vi "UHR-Fleezers Control (host) - 12.8.vi"() -> ()   [LabVIEW 2012] (continued)
          tunnel: [w4443 w4464] -> w4429
          tunnel: [w4442 w4463] -> w4428
          tunnel: w4427 -> [w4443 w4469]
          tunnel: w4426 -> [w4442 w4472]
          tunnel: w4423 -> [_ _]
          frame False {
            w4444 = TRUE ("AI to FIFO")
            n2524 = xnode "Read/Write Control"("FPGA VI Reference In"=w4448, "error in"=w4447, "AI to FIFO"=w4444, "APD to FIFO"=w4444, "Start scan (MCL)"=w4444) -> ("FPGA VI Reference Out"=w4446:T20, "error out"=w4445:errorcluster)
          }
          frame True {
            w4476 = TRUE ("AI to FIFO")
            n2525 = local read "Scan steps (MCL)"() -> (w4455:u64)
            n2526 = local read "Scan lines (y)"() -> (w4451:u64)
            n2527 = local read "Fast Scan Dir"() -> (w4462:bool)
            n2528 = local read "Actual MCL Inc (V)"() -> (w4452:dbl)
            n2529 = Decrement(x=w4451) -> (x-1=w4450:u64)
            n2530 = Decrement(x=w4455) -> (x-1=w4454:u64)
            n2531 = Multiply(x=w4452, y=w4450) -> (x*y=w4449:dbl)
            n2532 = Divide(x=w4449, y=2.0) -> (x/y=w4459:dbl)
            n2533 = Multiply(x=w4452, y=w4454) -> (x*y=w4453:dbl)
            n2534 = Divide(x=w4453, y=2.0) -> (x/y=w4458:dbl)
            n2535 = Select(t=w4458, s=w4462, f=w4459) -> (s? t:f=w4457:dbl)
            n2536 = Select(t=w4459, s=w4462, f=w4458) -> (s? t:f=w4461:dbl)
            n2537 = Subtract(x=w4469, y=w4461) -> (x-y=w4460:dbl)
            n2538 = Subtract(x=w4472, y=w4457) -> (x-y=w4456:dbl)
            n2539 = local read "2D or 1D Scan"() -> (w4474:bool)
            n2540 = Not(x=w4462) -> (.not. x?=w4468:bool)
            n2541 = Not(x=w4474) -> (.not. x?=w4470:bool)
            n2542 = And(x=w4462, y=w4470) -> (x .and. y?=w4471:bool)
            n2543 = And(x=w4470, y=w4468) -> (x .and. y?=w4473:bool)
            n2544 = Select(t=w4472, s=w4473, f=w4456) -> (s? t:f=w4463:dbl)
            n2545 = Select(t=w4469, s=w4471, f=w4460) -> (s? t:f=w4464:dbl)
            n2546 = call "Volt to I16.vi"("Voltage In"=w4464) -> ("I16 Voltage Out"=w4467:i16)
            n2547 = call "Volt to I16.vi"("Voltage In"=w4463) -> ("I16 Voltage Out"=w4466:i16)
            n2548 = xnode "Read/Write Control"("FPGA VI Reference In"=w4480, "error in"=w4479, "AI to FIFO"=w4476, "APD to FIFO"=w4476, "Start scan (MCL)"=w4476, "AO1"=w4467, "AO2"=w4466) -> ("FPGA VI Reference Out"=w4478:T20, "error out"=w4477:errorcluster)
          }
        }
        "Initial Y" <- w4429
        "Initial X" <- w4428
        n2549 = local write "Tab Control 6"(T3."Imaging" ("Tab Control 6")) -> ()
        "wait to reset values" <- w4430
      }
    }
    n2550 = local read "APD Elements/DMA read"() -> (w3570:u32)
    n2551 = local read "Trap AI Elements/DMA read"() -> (w3785:u32)
    n2552 = xnode "Get APD Data"("FPGA VI Reference In"=w3726, "error in"=w3725, "Number of Elements"=w3570, "Timeout (ms)"=-1) -> ("Data"=w3756:u32[], "Elements Remaining"=→"APD FIFO Elements Remaining":u32)  [unwired: 2 out]
    n2553 = local read "Trap Pos Elements/DMA read"() -> (w3722:u32)
    n2554 = xnode "Invoke Method"("FPGA VI Reference In"=w3726, "error in"=w3725, "Number of Elements"=w3722, "Timeout (ms)"=-1) -> ("Data"=w3686:u16[], "Elements Remaining"=→"Trap Pos FIFO El Remaining":u32)  [unwired: 2 out]
    n2555 = xnode "Get Trap Data"("FPGA VI Reference In"=w3726, "error in"=w3725, "Number of Elements"=w3785, "Timeout (ms)"=-1 ("Timeout")) -> ("FPGA VI Reference Out"=w3621:T20, "error out"=w3620:errorcluster, "Data"=w3687:i16[], "Elements Remaining"=w3903:u32)
    "FIFO El. Rem." <- w3903
    n2556 = local read "DMA Update Period (s)"() -> (w3786:dbl)
    n2557 = local read "Trap AI FIFO Depth"() -> (w3905:u32)
    n2558 = local read "Number of APDs"() -> (w3589:u8)
    n2559 = Decimate 1D Array(w3686) -> (w3683:u16[], w3685:u16[], w3684:u16[])
    n2560 = feedback #6(0.0) -> (w3715:dbl)
    n2561 = Add(x=w3786, y=w3715) -> (x+y=w3879:dbl)
    n2562 = feedback-in #6(w3879) -> ()
    n2563 = To Time Stamp(1:w3715) -> (0:w3714:timestamp)
    n2564 = Subtract(x=w3905, y=w3785) -> (x-y=w3904:u32)
    n2565 = To Unsigned Long Integer(number=w3683) -> (unsigned 32bit integer=w3682:u32[])
    n2566 = Join Numbers(hi=w3685, lo=w3684) -> ((hi.lo)=w3681:u32[])
    n2567 = Divide(x=w3903, y=w3904) -> (x/y=w3902:dbl)
    "Buffer Status" <- w3902
    n2568 = case "Deinterlace APD signals" shown="3, Default" w3589 {
      tunnel: [w3929 w3935] -> w3569
      tunnel: w3756 -> [w3930 w3934]
      tunnel: [w3928 w3933] -> w3568
      tunnel: [w3927 w3931] -> w3557
      frame 3, Default {
        n2569 = Decimate 1D Array "APD signals"(w3930) -> (w3929:u32[], w3928:u32[], w3927:u32[])
      }
      frame 2 {
        n2570 = Decimate 1D Array "APD signals"(w3934) -> (w3935:u32[], w3933:u32[])
        n2571 = Multiply(x=w3933, y=u32 0) -> (x*y=w3931:u32[])
      }
    }
    n2572 = Join Numbers(hi=w3682, lo=w3681) -> ((hi.lo)=w3675:u64[])
    n2573 = call "IR AOM word to freq - vec.vi"("Frequency Word In (double vec)"=w3675) -> ("Frequency Out"=w3721:dbl[])
    n2574 = Equal?(x=w3902, y=1.0) -> (x = y?=w3900:bool)
    n2575 = case "Alert buffer overflow" shown="True" w3900 {
      frame False {
      }
      frame True {
        n2576 = call <vilib>:"Beep.vi"() -> ()  [unwired: 3 in, 9 out]
        "Overflow (data lost)" <- TRUE ("Overflow (data lost)")
      }
    }
    n2577 = Decimate 1D Array(w3721) -> (w3720:dbl[], w3719:dbl[])
    n2578 = Build Array(w3720, w3719) -> (w3718:dbl[][])
    n2579 = Bundle(w3569, w3568, w3557) -> (w3573:cluster{u32[], u32[], u32[]})  [unwired: 1 in]
    n2580 = Build Array(w3569, w3568, w3557) -> (w3840:u32[][])
    n2581 = for {
      tunnel: w3569 -> [w3925] mode=indexing
      n2582 = call "Smart Buffer (DBL) 1.vi"("new element [write]"=w3925, "mode"=T21."write") -> ()  [unwired: 4 in, 6 out]
    }
    n2583 = local read "APD Integration Time (s)"() -> (w3584:dbl)
    n2584 = To Double Precision Float(number=w3840) -> (double precision float=w3841:dbl[][])
    n2585 = feedback #7 "APD3"(w3557) -> (w3558:u32[])
    n2586 = feedback #8 "APD2"(w3568) -> (w3744:u32[])
    n2587 = feedback #9 "APD1"(w3569) -> (w3839:u32[])
    n2588 = Build Array (concatenate)(w3744, w3568) -> (w3743:u32[])
    n2589 = Build Array (concatenate)(w3558, w3557) -> (w3556:u32[])
    n2590 = Build Array (concatenate)(w3839, w3569) -> (w3836:u32[])
    n2591 = for {
      tunnel: w3568 -> [w3924] mode=indexing
      n2592 = call "Smart Buffer (DBL) 2.vi"("new element [write]"=w3924, "mode"=T21."write") -> ()  [unwired: 4 in, 6 out]
    }
    n2593 = Array Size(array=w3836) -> (size(s)=w3833:i32)
    n2594 = Array Size(array=w3569) -> (size(s)=w3835:i32)
    n2595 = Multiply(x=w3835, y="APD Ave N") -> (x*y=w3834:dbl)
    n2596 = Greater?(x=w3833, y=w3834) -> (0:w3837:bool)
    n2597 = Bundle("APD 1", "APD 2", "APD 3") -> (w3873:cluster{string, string, string})  [unwired: 1 out]
    n2598 = local read "Trap Sets"() -> (w3784:u32)
    n2599 = case shown="True" w3837 {
      tunnel: w3836 -> [w4236 w4245]
      tunnel: [w4236 w4243] -> w3791
      tunnel: w3834 -> [_ w4238]
      tunnel: w3833 -> [_ w4244]
      tunnel: w3743 -> [w4235 w4242]
      tunnel: [w4235 w4241] -> w3741
      tunnel: w3556 -> [w4234 w4240]
      tunnel: [w4234 w4237] -> w3585
      frame False {
      }
      frame True {
        n2600 = Subtract(x=w4244, y=w4238) -> (x-y=w4239:dbl)
        n2601 = Array Subset "APD3"(array=w4240, index=w4239, length=w4238) -> (w4237:u32[])
        n2602 = Array Subset "APD2"(array=w4242, index=w4239, length=w4238) -> (w4241:u32[])
        n2603 = Array Subset "APD1"(array=w4245, index=w4239, length=w4238) -> (w4243:u32[])
      }
    }
    n2604 = feedback-in #7(w3585) -> ()
    n2605 = feedback-in #8(w3741) -> ()
    n2606 = feedback-in #9(w3791) -> ()
    n2607 = Cluster To Array(cluster=w3873) -> (array=w3870:string[])
    n2608 = for "APD" {
      tunnel: w3841 -> [w4492] mode=indexing
      tunnel: w3584 -> [w4499]
      tunnel: [w4495] -> w3745 mode=indexing
      tunnel: "APD Disp. Scale" -> [w4496]
      tunnel: w3870 -> [w4494] mode=indexing
      tunnel: "APD Disp. Downsample" -> [w4490]
      tunnel: [w4493] -> w3869
      workers-P: _ -> [_]
      tunnel: w3714 -> [w4489]
      n2609 = call "integrate 1D array interval - double.vi"("Ave N"=w4490, "Array In"=w4492) -> ("Array Out"=w4491:dbl[])  [unwired: 1 out]
      n2610 = Multiply(x=w4499, y=w4490) -> (x*y=w4493:dbl)
      n2611 = Divide(x=w4491, y=w4496) -> (x/y=w4497:dbl[])
      n2612 = Bundle By Name("t0"=w4489, "Y"=w4497, "dt"=w4493) -> (w4498:waveform(dbl))  [unwired: 1 out]
      n2613 = Set Waveform Attribute(5:w4494, 6:"NI_ChannelName" ("name"), 7:w4498) -> (3:w4495:waveform(dbl))  [unwired: 1 in, 2 out]
    }
    "APD Display Period (s)" <- w3869
    n2614 = Reciprocal(x=w3869) -> (1/x=→"APD Display Freq. (Hz)":dbl)
    n2615 = case "Deinterlace trap data, average down PSD" shown="2" w3784 {
      tunnel: w3687 -> [w4517 w4582]
      tunnel: [w4514 w4579] -> w3777
      tunnel: [w4517 w4581] -> w3678
      tunnel: "Detector Type" -> [w4516 w4577]
      tunnel: [w4515 w4580] -> w3776
      tunnel: [w4513 w4578] -> w3877
      frame 1, Default {
        n2616 = Divide(x=w4517, y=3276.7) -> (x/y=w4518:dbl[])
        n2617 = Decimate 1D Array(w4518) -> (w4527:dbl[], w4526:dbl[], w4525:dbl[], w4524:dbl[], w4523:dbl[], w4522:dbl[], w4521:dbl[], w4520:dbl[])
        n2618 = case shown="\"IR-QPD + PSD + FB-QPD position\"" w4516 {
          tunnel: w4527 -> [w4551 w4576]
          tunnel: w4526 -> [w4550 w4575]
          tunnel: w4525 -> [w4535 w4553]
          tunnel: w4524 -> [w4536 w4563]
          tunnel: w4523 -> [w4549 w4574]
          tunnel: w4522 -> [w4548 w4573]
          tunnel: w4521 -> [w4532 w4554]
          tunnel: w4520 -> [w4531 w4552]
          tunnel: [w4530 w4560] -> w4515
          tunnel: [w4529 w4559] -> w4514
          tunnel: [w4528 w4558] -> w4513
          frame "IR-QPD + PSD + FB-QPD", Default {
            w4528 = 0  # Channel pattern
            n2619 = Divide(x=w4551, y=w4536) -> (x/y=w4538:dbl[])
            n2620 = Divide(x=w4550, y=w4536) -> (x/y=w4537:dbl[])
            n2621 = Divide(x=w4549, y=w4532) -> (x/y=w4534:dbl[])
            n2622 = Divide(x=w4548, y=w4531) -> (x/y=w4533:dbl[])
            n2623 = Build Array(w4538, w4537, w4536, w4535, w4534, w4533, w4532, w4531) -> (w4529:dbl[][])
            n2624 = Bundle("T1 Y", "T1 X", "T1 Sum", "FB Sum", "PSD Y", "PSD X", "PSD Y Sum", "PSD X Sum") -> (w4547:T44)  [unwired: 1 out]
            n2625 = Cluster To Array(cluster=w4547) -> (array=w4530:string[])
          }
          frame "IR-QPD + PSD + FB-QPD position" {
            w4558 = 3  # Channel pattern
            n2626 = Negate(x=w4554) -> (-x=w4555:dbl[])
            n2627 = Divide(x=w4576, y=w4563) -> (x/y=w4565:dbl[])
            n2628 = Divide(x=w4575, y=w4563) -> (x/y=w4564:dbl[])
            n2629 = Divide(x=w4574, y=w4554) -> (x/y=w4562:dbl[])
            n2630 = Divide(x=w4573, y=w4555) -> (x/y=w4561:dbl[])
            n2631 = Build Array(w4565, w4564, w4563, w4552, w4553, w4562, w4561, w4554) -> (w4559:dbl[][])
            n2632 = Bundle("T1 Y", "T1 X", "T1 Sum", "FB X", "FB Sum", "PSD Y", "PSD X", "PSD Y Sum") -> (w4572:T44)  [unwired: 1 out]
            n2633 = Cluster To Array(cluster=w4572) -> (array=w4560:string[])
          }
        }
      }
      frame 2 {
        n2634 = case shown="\"IR-QPD + PSD + FB-QPD X position\", Default" w4577 {
          tunnel: w4582 -> [w4644 w4716 w4787]
          tunnel: [w4583 w4707 w4718] -> w4581
          tunnel: [w4610 w4698 w4765] -> w4580
          tunnel: [w4609 w4661 w4732] -> w4579
          tunnel: [w4603 w4696 w4763] -> w4578
          frame "IR-QPD + PSD + FB-QPD" {
            w4603 = 1  # Channel pattern
            # "time average x2 the 4th signal and the 4 psd signals (detection laser)"
            # "deinterlace 3 signals from qpd"
            n2635 = Decimate 1D Array(w4644) -> (w4643:i16[], w4642:i16[], w4608:i16[], w4641:i16[], w4631:i16[], w4629:i16[], w4628:i16[], w4626:i16[])
            n2636 = Decimate 1D Array(w4608) -> (w4607:i16[], w4606:i16[])
            n2637 = Decimate 1D Array(w4643) -> (w4640:i16[], w4612:i16[])
            n2638 = Decimate 1D Array(w4642) -> (w4639:i16[], w4637:i16[])
            n2639 = Decimate 1D Array(w4641) -> (w4638:i16[], w4636:i16[])
            n2640 = call "downsample 1D array - double.vi"("Ave N"=2.0, "Array In"=w4631) -> ("Array Out"=w4630:dbl[])  [unwired: 1 out]
            n2641 = call "downsample 1D array - double.vi"("Ave N"=2.0, "Array In"=w4629) -> ("Array Out"=w4611:dbl[])  [unwired: 1 out]
            n2642 = call "downsample 1D array - double.vi"("Ave N"=2.0, "Array In"=w4628) -> ("Array Out"=w4627:dbl[])  [unwired: 1 out]
            n2643 = call "downsample 1D array - double.vi"("Ave N"=2.0, "Array In"=w4626) -> ("Array Out"=w4625:dbl[])  [unwired: 1 out]
            n2644 = Interleave 1D Arrays(w4640, w4639, w4638, w4612, w4637, w4636, w4607, w4606, w4630, w4611, w4627, w4625) -> (w4624:dbl[])
            n2645 = Divide(x=w4624, y=3276.7) -> (x/y=w4623:dbl[])
            n2646 = Decimate 1D Array(w4623) -> (w4622:dbl[], w4621:dbl[], w4620:dbl[], w4619:dbl[], w4618:dbl[], w4617:dbl[], w4605:dbl[], w4604:dbl[], w4616:dbl[], w4615:dbl[], w4614:dbl[], w4613:dbl[])
            n2647 = Divide(x=w4622, y=w4620) -> (x/y=w4590:dbl[])
            n2648 = Divide(x=w4621, y=w4620) -> (x/y=w4589:dbl[])
            n2649 = Divide(x=w4619, y=w4617) -> (x/y=w4588:dbl[])
            n2650 = Divide(x=w4618, y=w4617) -> (x/y=w4587:dbl[])
            n2651 = Divide(x=w4616, y=w4614) -> (x/y=w4586:dbl[])
            n2652 = Divide(x=w4615, y=w4613) -> (x/y=w4585:dbl[])
            n2653 = Build Array(w4590, w4589, w4620, w4588, w4587, w4617, w4605, w4604, w4586, w4585, w4614, w4613) -> (w4609:dbl[][])
            n2654 = Bundle("T1 Y", "T1 X", "T1 Sum", "T2 Y", "T2 X", "T2 Sum", "T1 FB Sum", "T2 FB Sum", "PSD Y", "PSD X", "PSD Y Sum", "PSD X Sum") -> (w4591:T45)  [unwired: 1 out]
            n2655 = To Word Integer(number=w4624) -> (16bit integer=w4583:i16[])
            n2656 = Cluster To Array(cluster=w4591) -> (array=w4610:string[])
          }
          frame "IR-QPD + PSD + FB-QPD X position", Default {
            w4696 = 2  # Channel pattern
            # "time average x2 the 3 psd signals (detection laser)"
            # "deinterlace 3 signals from qpds"
            n2657 = Decimate 1D Array(w4716) -> (w4715:i16[], w4714:i16[], w4697:i16[], w4713:i16[], w4659:i16[], w4656:i16[], w4653:i16[], w4684:i16[])
            n2658 = Select(t=i16 -1, s="Flip X Sign", f=i16 1) -> (s? t:f=w4649:i16)
            n2659 = Multiply(x=w4714, y=w4649) -> (x*y=w4650:i16[])
            n2660 = Decimate 1D Array(w4697) -> (w4682:i16[], w4680:i16[])
            n2661 = Decimate 1D Array(w4715) -> (w4712:i16[], w4699:i16[])
            n2662 = Decimate 1D Array(w4650) -> (w4711:i16[], w4709:i16[])
            n2663 = Decimate 1D Array(w4713) -> (w4710:i16[], w4708:i16[])
            n2664 = Decimate 1D Array(w4684) -> (w4683:i16[], w4681:i16[])
            n2665 = call "downsample 1D array - I16.vi"("Ave N"=2.0, "Array In"=w4659) -> ("Array Out"=w4657:i16[])  [unwired: 1 in]
            n2666 = call "downsample 1D array - I16.vi"("Ave N"=2.0, "Array In"=w4653) -> ("Array Out"=w4651:i16[])  [unwired: 1 in]
            n2667 = call "downsample 1D array - I16.vi"("Ave N"=2.0, "Array In"=w4656) -> ("Array Out"=w4654:i16[])  [unwired: 1 in]
            n2668 = Interleave 1D Arrays(w4712, w4711, w4710, w4699, w4709, w4708, w4683, w4682, w4681, w4680, w4657, w4654, w4651) -> (w4707:i16[])
            n2669 = Divide(x=w4707, y=3276.7) -> (x/y=w4706:dbl[])
            n2670 = Decimate 1D Array(w4706) -> (w4705:dbl[], w4704:dbl[], w4703:dbl[], w4702:dbl[], w4701:dbl[], w4700:dbl[], w4672:dbl[], w4670:dbl[], w4669:dbl[], w4667:dbl[], w4666:dbl[], w4665:dbl[], w4662:dbl[])
            n2671 = Negate(x=w4662) -> (-x=w4660:dbl[])
            n2672 = Divide(x=w4666, y=w4662) -> (x/y=w4664:dbl[])
            n2673 = Divide(x=w4665, y=w4660) -> (x/y=w4663:dbl[])
            n2674 = Divide(x=w4705, y=w4703) -> (x/y=w4688:dbl[])
            n2675 = Divide(x=w4704, y=w4703) -> (x/y=w4687:dbl[])
            n2676 = Divide(x=w4702, y=w4700) -> (x/y=w4686:dbl[])
            n2677 = Divide(x=w4701, y=w4700) -> (x/y=w4685:dbl[])
            n2678 = Divide(x=w4672, y=w4670) -> (x/y=w4671:dbl[])
            n2679 = Divide(x=w4669, y=w4667) -> (x/y=w4668:dbl[])
            n2680 = Build Array(w4688, w4687, w4703, w4686, w4685, w4700, w4671, w4670, w4668, w4667, w4664, w4663, w4662) -> (w4661:dbl[][])
            n2681 = Bundle("T1 Y", "T1 X", "T1 Sum", "T2 Y", "T2 X", "T2 Sum", "T1 FB X", "T1 FB Sum", "T2 FB X", "T2 FB Sum", "PSD Y", "PSD X", "PSD Y Sum") -> (w4689:T46)  [unwired: 1 out]
            n2682 = Cluster To Array(cluster=w4689) -> (array=w4698:string[])
          }
          frame "IR-QPD + PSD + FB-QPD XY positions" {
            w4763 = 4  # Channel pattern
            # "time average x2 the 3 psd signals (detection laser)"
            # "deinterlace 3 signals from qpds"
            n2683 = Decimate 1D Array(w4787) -> (w4786:i16[], w4785:i16[], w4764:i16[], w4784:i16[], w4730:i16[], w4776:i16[], w4775:i16[], w4752:i16[])
            n2684 = Decimate 1D Array "Feedback Sum"(w4764) -> (w4748:i16[], w4746:i16[])
            n2685 = Decimate 1D Array "QPD Y"(w4786) -> (w4783:i16[], w4766:i16[])
            n2686 = Decimate 1D Array "QPD X"(w4785) -> (w4782:i16[], w4780:i16[])
            n2687 = Decimate 1D Array "Feedback Y"(w4730) -> (w4729:i16[], w4728:i16[])
            n2688 = Decimate 1D Array "QPD Sum"(w4784) -> (w4781:i16[], w4779:i16[])
            n2689 = Decimate 1D Array "Feedback X"(w4752) -> (w4749:i16[], w4747:i16[])
            n2690 = call "downsample 1D array - double.vi"("Ave N"=2.0, "Array In"=w4776) -> ("Array Out"=w4751:dbl[])  [unwired: 1 out]
            n2691 = call "downsample 1D array - double.vi"("Ave N"=2.0, "Array In"=w4775) -> ("Array Out"=w4750:dbl[])  [unwired: 1 out]
            n2692 = Interleave 1D Arrays(w4783, w4782, w4781, w4766, w4780, w4779, w4729, w4749, w4748, w4728, w4747, w4746, w4751, w4750) -> (w4774:dbl[])
            n2693 = Divide(x=w4774, y=3276.7) -> (x/y=w4773:dbl[])
            n2694 = Decimate 1D Array(w4773) -> (w4772:dbl[], w4771:dbl[], w4770:dbl[], w4769:dbl[], w4768:dbl[], w4767:dbl[], w4725:dbl[], w4739:dbl[], w4723:dbl[], w4724:dbl[], w4737:dbl[], w4721:dbl[], w4735:dbl[], w4733:dbl[])
            n2695 = Negate(x=w4733) -> (-x=w4731:dbl[])
            n2696 = Divide(x=w4735, y=w4731) -> (x/y=w4734:dbl[])
            n2697 = Divide(x=w4724, y=w4721) -> (x/y=w4720:dbl[])
            n2698 = Divide(x=w4725, y=w4723) -> (x/y=w4722:dbl[])
            n2699 = Divide(x=w4772, y=w4770) -> (x/y=w4756:dbl[])
            n2700 = Divide(x=w4771, y=w4770) -> (x/y=w4755:dbl[])
            n2701 = Divide(x=w4769, y=w4767) -> (x/y=w4754:dbl[])
            n2702 = Divide(x=w4768, y=w4767) -> (x/y=w4753:dbl[])
            n2703 = Divide(x=w4739, y=w4723) -> (x/y=w4738:dbl[])
            n2704 = Divide(x=w4737, y=w4721) -> (x/y=w4736:dbl[])
            n2705 = Build Array(w4756, w4755, w4770, w4754, w4753, w4767, w4722, w4738, w4723, w4720, w4736, w4721, w4734, w4733) -> (w4732:dbl[][])
            n2706 = Bundle("T1 Y", "T1 X", "T1 Sum", "T2 Y", "T2 X", "T2 Sum", "T1 FB Y", "T1 FB X", "T1 FB Sum", "T2 FB Y", "T2 FB X", "T2 FB Sum", "PSD X", "PSD Y Sum") -> (w4719:T47)  [unwired: 1 out]
            n2707 = To Word Integer(number=w4774) -> (16bit integer=w4718:i16[])
            n2708 = Cluster To Array(cluster=w4719) -> (array=w4765:string[])
          }
        }
      }
    }
    "AI labels" <- w3776
    n2709 = local read "APD Integration Time (s)"() -> (w3751:dbl)
    n2710 = Array Size(array=w3791) -> (size(s)=w3832:i32)
    n2711 = call <vilib>:"Std Deviation and Variance.vi"("X"=w3741) -> ("standard deviation"=w3740:dbl)  [unwired: 1 in, 2 out]
    n2712 = Add Array Elements(numeric array=w3741) -> (sum=w3742:u32)
    n2713 = Add Array Elements(numeric array=w3791) -> (sum=w3842:u32)
    n2714 = call <vilib>:"Std Deviation and Variance.vi"("X"=w3791) -> ("standard deviation"=w3790:dbl)  [unwired: 1 in, 2 out]
    n2715 = Divide(x=w3740, y=w3584) -> (x/y=w3737:dbl)
    "Rate sigma (Hz) 2" <- w3737
    n2716 = Multiply(x=w3584, y=w3832) -> (x*y=w3586:dbl)
    "Int. Time (s)" <- w3586
    n2717 = Divide(x=w3742, y=w3586) -> (x/y=w3738:dbl)
    "APD 2 Rate (Hz)" <- w3738
    n2718 = Multiply(x="APD Disp. Scale", y=w3745) -> (x*y=w3753:waveform(dbl)[])
    n2719 = Divide(x=w3842, y=w3586) -> (x/y=w3788:dbl)
    "APD 1 Rate (Hz)" <- w3788
    n2720 = Divide(x=w3790, y=w3584) -> (x/y=w3789:dbl)
    "Rate sigma (Hz)" <- w3789
    n2721 = Divide(x=w3737, y=w3738) -> (x/y=→"Sigma/Mean 2":dbl)
    n2722 = Multiply(x="APD Disp. Downsample", y=w3751) -> (x*y=w3749:dbl)
    n2723 = Divide(x=w3789, y=w3788) -> (x/y=→"Sigma/Mean":dbl)
    n2724 = Divide(x=w3753, y=w3749) -> (x/y=w3576:waveform(dbl)[])
    n2725 = Index Array(array=w3576, index=0) -> (element=w3734:waveform(dbl))
    n2726 = Index Array(array=w3576, index=1) -> (element=w3732:waveform(dbl))
    n2727 = Index Array(array=w3576, index=2) -> (element=w3578:waveform(dbl))
    n2728 = Subtract(x=w3734, y="APD 1 Offset") -> (x-y=w3730:waveform(dbl))
    n2729 = Subtract(x=w3732, y="APD 2 Offset") -> (x-y=w3729:waveform(dbl))
    n2730 = Subtract(x=w3578, y="APD 3 Offset") -> (x-y=w3575:waveform(dbl))
    n2731 = Add Array Elements(numeric array=w3585) -> (sum=w3588:u32)
    n2732 = call <vilib>:"Std Deviation and Variance.vi"("X"=w3585) -> ("standard deviation"=w3587:dbl)  [unwired: 1 in, 2 out]
    n2733 = Build Array(w3730, w3729, w3575) -> (→"APD Chart":waveform(dbl)[])
    n2734 = Divide(x=w3588, y=w3586) -> (x/y=w3582:dbl)
    "APD 3 Rate (Hz)" <- w3582
    n2735 = Divide(x=w3587, y=w3584) -> (x/y=w3583:dbl)
    "Rate sigma (Hz) 3" <- w3583
    n2736 = Divide(x=w3583, y=w3582) -> (x/y=→"Sigma/Mean 3":dbl)
    n2737 = local read "Data Period (s)"() -> (w3637:dbl)
    n2738 = local read "BD 1 Frequency 2 (MHz)"() -> (w3670:dbl)
    n2739 = local read "BD 1 Frequency 1 (MHz)"() -> (w3671:dbl)
    n2740 = Decimate 1D Array(w3678) -> (w3702:i16[], w3701:i16[], w3699:i16[], w3698:i16[])  [unwired: 9 out]
    n2741 = Multiply(x=w3637, y="Trap Pos. Disp. Downsample") -> (x*y=w3635:dbl)
    n2742 = Divide(x=w3702, y=w3701) -> (x/y=w3703:dbl[])
    n2743 = Divide(x=w3699, y=w3698) -> (x/y=w3700:dbl[])
    n2744 = local read "AOM X Cal (nm/MHz)"() -> (w3668:dbl)
    n2745 = Split 1D Array(array=w3703, index="N El. to Ave.") -> (second subarray=w3706:dbl[])  [unwired: 1 out]
    n2746 = Split 1D Array(array=w3700, index="N El. to Ave.") -> (second subarray=w3705:dbl[])  [unwired: 1 out]
    n2747 = Multiply(x=w3637, y="Trap Disp. Downsample") -> (x*y=w3716:dbl)
    "Display Period (s)" <- w3716
    n2748 = for "Trap AI" {
      tunnel: [w4512] -> w3563 mode=indexing
      tunnel: w3714 -> [w4503]
      tunnel: "Trap Disp. Downsample" -> [w4510]
      tunnel: w3777 -> [w4508] mode=indexing
      tunnel: w3637 -> [w4507]
      tunnel: w3776 -> [w4506] mode=indexing
      tunnel: [w4505] -> w3748 mode=indexing
      tunnel: w3716 -> [w4504]
      workers-P: _ -> [_]
      n2749 = Bundle By Name("Y"=w4508, "dt"=w4507) -> (w4509:waveform(dbl))  [unwired: 1 out]
      n2750 = Set Waveform Attribute(5:w4506, 6:"NI_ChannelName" ("name"), 7:w4509) -> (3:w4505:waveform(dbl))  [unwired: 1 in, 2 out]
      n2751 = call "downsample 1D array - double.vi"("Ave N"=w4510, "Array In"=w4508) -> ("Array Out"=w4511:dbl[])  [unwired: 1 out]
      n2752 = Bundle By Name(cluster=w4505, "t0"=w4503, "Y"=w4511, "dt"=w4504) -> (w4512:waveform(dbl))
    }
    n2753 = Bundle("BD 1 Frequency 1 (MHz)"=w3671, "BD 1 Frequency 2 (MHz)"=w3670) -> (w3672:T48)  [unwired: 1 out]
    n2754 = call-poly <vilib>:"Mean.vi"("X"=w3705) -> ("mean"=w3693:dbl)  [unwired: 1 out]
    n2755 = call-poly <vilib>:"Mean.vi"("X"=w3706) -> ("mean"=w3694:dbl)  [unwired: 1 out]
    n2756 = Reciprocal(x=w3716) -> (1/x=→"Trap Disp. Freq. (Hz)":dbl)
    n2757 = Cluster To Array(cluster=w3672) -> (array=w3669:dbl[])
    n2758 = local read "Trap X AI1 (DMA)"() -> (w3704:T13)
    n2759 = local read "Data points/scans (MCL)"() -> (w3852:dbl)
    n2760 = To Fixed-Point(number=w3693) -> (fixed-point=w3691:fxp<+/-,16,1>)  [unwired: 1 in]
    n2761 = To Fixed-Point(number=w3694) -> (fixed-point=w3692:fxp<+/-,16,1>)  [unwired: 1 in]
    n2762 = Bundle("Trap 1 Pos.", "Trap 2 Pos.") -> (w3713:cluster{string, string})  [unwired: 1 out]
    n2763 = Bundle By Name(cluster=w3704, "Set 1"=w3692, "Set 2"=w3691) -> (→"Trap X AI1 (DMA)":T13)
    n2764 = Cluster To Array(cluster=w3713) -> (array=w3710:string[])
    n2765 = Unbundle(w3573) -> (w3574:u32[])  [unwired: 2 out]
    n2766 = Select(t=-1.0, s="Negate Y Axis", f=1.0) -> (s? t:f=w3654:dbl)
    n2767 = for "Trap Position" {
      tunnel: w3718 -> [w4095] mode=indexing
      tunnel: "Trap Pos. Disp. Downsample" -> [w4094]
      tunnel: w3635 -> [w4092]
      tunnel: w3714 -> [w4091]
      tunnel: w3710 -> [w4089] mode=indexing
      tunnel: [w4088] -> w3624 mode=indexing
      tunnel: w3669 -> [w4086] mode=indexing
      tunnel: w3668 -> [w4084]
      tunnel: w3654 -> [w4083]
      n2768 = call "downsample 1D array - double.vi"("Ave N"=w4094, "Array In"=w4095) -> ("Array Out"=w4093:dbl[])  [unwired: 1 out]
      n2769 = Subtract(x=w4093, y=w4086) -> (x-y=w4087:dbl[])
      n2770 = Multiply(x=w4084, y=w4087) -> (x*y=w4085:dbl[])
      n2771 = Multiply(x=w4083, y=w4085) -> (x*y=w4082:dbl[])
      n2772 = Bundle By Name("Y"=w4082, "dt"=w4092, "t0"=w4091) -> (w4090:waveform(dbl))  [unwired: 1 out]
      n2773 = Set Waveform Attribute(5:w4089, 6:"NI_ChannelName" ("name"), 7:w4090) -> (3:w4088:waveform(dbl))  [unwired: 1 in, 2 out]
    }
    n2774 = To Double Precision Float(number=w3574) -> (double precision float=w3774:dbl[])
    n2775 = local read "Display Period (s)"() -> (w3765:dbl)
    n2776 = Increment(x=w3852) -> (x+1=w3853:dbl)
    n2777 = Index Array(array=w3624, index=0) -> (element=w3628:waveform(dbl))
    n2778 = Index Array(array=w3624, index=1) -> (element=w3623:waveform(dbl))
    n2779 = feedback #10(w3853) -> (w3856:dbl)
    n2780 = Select(t=0, s=w3843, f=w3856) -> (s? t:f=w3849:dbl)
    n2781 = Array Size(array=w3774) -> (size(s)=w3855:i32)
    n2782 = Build Array (concatenate)(w3745, w3563) -> (w3554:waveform(dbl)[])
    "All Signals" <- w3554
    n2783 = Add(x=w3855, y=w3849) -> (x+y=w3850:dbl)
    n2784 = Unbundle By Name(w3628) -> ("Y"=w3629:dbl[])
    n2785 = Divide(x="Bead Sep. Int. Time (s)", y=w3765) -> (x/y=w3664:dbl)
    n2786 = Add(x=w3629, y="FB Trap Pos Offset") -> (x+y=w3627:dbl[])
    "T1 x pos data" <- w3627
    n2787 = Greater?(x=w3850, y=w3852) -> (0:w3851:bool)
    n2788 = feedback #11(w3627) -> (w3666:dbl[])
    n2789 = Build Array (concatenate)(w3627, w3666) -> (w3665:dbl[])
    n2790 = Bundle By Name(cluster=w3628, "Y"=w3627) -> (w3626:waveform(dbl))
    n2791 = Select(t=w3849, s=w3851, f=w3850) -> (s? t:f=w3848:dbl)
    n2792 = feedback-in #10(w3848) -> ()
    n2793 = local read "MCL Scanning"() -> (w3846:bool)
    n2794 = Bundle(w3626, w3623) -> (w3622:cluster{waveform(dbl), waveform(dbl)})  [unwired: 1 out]
    n2795 = Index Array(array=w3563, index="index 1") -> (element=w3562:waveform(dbl))
    n2796 = Index Array(array=w3563, index="index 2") -> (element=w3567:waveform(dbl))
    n2797 = Split 1D Array(array=w3665, index=w3664) -> (first subarray=w3658:dbl[])  [unwired: 1 out]
    n2798 = feedback-in #11(w3658) -> ()
    n2799 = Unbundle By Name(w3562) -> ("Y"=w3561:dbl[])
    n2800 = Unbundle By Name(w3567) -> ("Y"=w3566:dbl[])
    n2801 = Not(x=w3851) -> (.not. x?=w3845:bool)
    n2802 = Cluster To Array(cluster=w3622) -> (array=w3598:waveform(dbl)[])
    "Trap Positions" <- w3598
    n2803 = call-poly <vilib>:"Mean.vi"("X"=w3658) -> ("mean"=w3657:dbl)  [unwired: 1 out]
    "Mean T1 Position (nm)" <- w3657
    n2804 = Subtract(x=w3658, y=w3657) -> (x-y=w3663:dbl[])
    n2805 = Square(x=w3663) -> (x^2=w3662:dbl[])
    n2806 = And(x=w3845, y=w3846) -> (x .and. y?=w3847:bool)
    n2807 = call-poly <vilib>:"Mean.vi"("X"=w3662) -> ("mean"=w3661:dbl)  [unwired: 1 out]
    n2808 = call-poly <vilib>:"Mean.vi"("X"=w3561) -> ("mean"=→"Trap 1 sum mean":dbl)  [unwired: 1 out]
    n2809 = call-poly <vilib>:"Mean.vi"("X"=w3566) -> ("mean"=→"Trap 2 sum mean":dbl)  [unwired: 1 out]
    n2810 = Square Root(x=w3661) -> (sqrt(x)=w3660:dbl)
    n2811 = Or(x=w3847, y=w3843) -> (x .or. y?=w3844:bool)
    n2812 = case shown="True" "X or Y?" {
      tunnel: w3554 -> [w3912 w3920]
      tunnel: [w3913 w3919] -> w3553
      tunnel: [w3911 w3918] -> w3552
      tunnel: ["T1 Y" ("Label.Text") "T1 X" ("Label.Text")] -> w3551
      tunnel: ["T2 Y" ("Label.Text") "T2 X" ("Label.Text")] -> w3550
      frame False {
        n2813 = Index Array(array=w3912, index=3) -> (element=w3913:waveform(dbl))
        n2814 = Index Array(array=w3912, index=6) -> (element=w3911:waveform(dbl))
      }
      frame True {
        n2815 = Index Array(array=w3920, index=4) -> (element=w3919:waveform(dbl))
        n2816 = Index Array(array=w3920, index=7) -> (element=w3918:waveform(dbl))
      }
    }
    n2817 = Equal?(x="Tab Control 6", y=T38."High Res Display") -> (x = y?=w3780:bool)
    n2818 = Multiply(x=10.0, y=w3660) -> (x*y=→"Trap 1 Position RMS (A)":dbl)
    n2819 = case "For displaying the high resolution display (no downsampling)" shown="True" w3780 {
      tunnel: w3748 -> [_ w4115]
      frame False {
      }
      frame True {
        n2820 = Index Array(array=w4115, index="High Res. Display") -> (element=w4116:waveform(dbl))
        n2821 = call <vilib>:"Std Deviation and Variance.vi"("X"=w4116) -> ("mean"=w4123:dbl, "standard deviation"=w4128:dbl)  [unwired: 1 in, 1 out]
        "Mean Intensity" <- w4123
        "Sigma" <- w4128
        n2822 = Subtract(x=w4116, y=w4123) -> (x-y=w4122:waveform(dbl))
        n2823 = Select(t=w4122, s="Subtract mean", f=w4116) -> (s? t:f=→"1 Channel":waveform(dbl))
        n2824 = Divide(x=w4128, y=w4123) -> (x/y=→"Sigma/Mean":dbl)
        n2825 = feedback #12(1) -> (w4117:i32)
        n2826 = Greater Or Equal?(x=w4117, y="Slow mean N ave.") -> (x >= y?=w4130:bool)
        n2827 = Increment(x=w4117) -> (x+1=w4132:i32)
        n2828 = Select(t=1, s=w4130, f=w4132) -> (s? t:f=w4119:i32)
        n2829 = feedback-in #12(w4119) -> ()
        n2830 = feedback #13() -> (w4120:waveform(dbl))  [unwired: 1 out]
        n2831 = case shown="Default" w4117 {
          tunnel: [w4135 w4138] -> w4121
          tunnel: w4120 -> [w4137 _]
          tunnel: w4116 -> [w4136 w4138]
          frame Default {
            n2832 = call-poly <vilib>:"Append Waveforms.vi"("waveform B"=w4136, "waveform A"=w4137) -> ("waveform out"=w4135:waveform(dbl))  [unwired: 1 in, 8 out]
          }
          frame 1 {
          }
        }
        n2833 = feedback-in #13(w4121) -> ()
        n2834 = case shown="True" w4130 {
          tunnel: w4121 -> [_ w4134]
          frame False {
          }
          frame True {
            n2835 = call-poly <vilib>:"Mean.vi"("X"=w4134) -> ("mean"=→"Slow mean":dbl)  [unwired: 1 out]
          }
        }
      }
    }
    n2836 = case "For plotting results of scanning MCL (fluorescence and detection laser images)" shown="True" w3844 {
      tunnel: w3843 -> [_ w4253]
      tunnel: w3852 -> [_ _]
      tunnel: w3748 -> [_ w4380]
      tunnel: w3727 -> [_ w4288]
      tunnel: w3573 -> [_ w4259]
      frame False {
      }
      frame True {
        w4269 = u32 0 items=["Horizontal", "Vertical", "Central", "1st Diagonal", "2nd Diagonal"] ("Type of Symmetry")
        w4295 = u32 0 items=["Horizontal", "Vertical", "Central", "1st Diagonal", "2nd Diagonal"] ("Type of Symmetry")
        w4319 = u32 0 items=["Horizontal", "Vertical", "Central", "1st Diagonal", "2nd Diagonal"] ("Type of Symmetry")
        w4322 = u32 0 items=["Horizontal", "Vertical", "Central", "1st Diagonal", "2nd Diagonal"] ("Type of Symmetry")
        w4351 = u32 0 items=["Horizontal", "Vertical", "Central", "1st Diagonal", "2nd Diagonal"] ("Type of Symmetry")
        n2837 = Unbundle(w4259) -> (w4258:u32[], w4256:u32[], w4254:u32[])
        n2838 = To Double Precision Float(number=w4258) -> (double precision float=w4257:dbl[])
        n2839 = To Double Precision Float(number=w4256) -> (double precision float=w4255:dbl[])
        n2840 = To Double Precision Float(number=w4254) -> (double precision float=w4247:dbl[])
        n2841 = Index Array(array=w4380, index=10) -> (element=w4386:waveform(dbl))
        n2842 = Index Array(array=w4380, index=11) -> (element=w4383:waveform(dbl))
        n2843 = local read "Cycles/step (MCL)"() -> (w4336:u64)
        n2844 = Index Array(array=w4380, index="Channel") -> (element=w4382:waveform(dbl))
        n2845 = Unbundle(w4288) -> ("New Image"=w4287:T2, "New Image"=w4286:T2, "New Image"=w4260:T2, "New Image"=w4261:T2, "New Image"=w4262:T2)
        n2846 = local read "Scan steps (MCL)"() -> (w4249:u64)
        n2847 = Unbundle By Name(w4386) -> ("Y"=w4338:dbl[])
        n2848 = Unbundle By Name(w4383) -> ("Y"=w4340:dbl[])
        n2849 = local read "Scan lines (y)"() -> (w4250:u64)
        n2850 = local read "N APD Samp/step"() -> (w4252:dbl)
        n2851 = Unbundle By Name(w4382) -> ("Y"=w4345:dbl[])
        n2852 = call "downsample 1D array - double.vi"("Ave N"=w4336, "Array In"=w4338) -> ("Array Out"=w4337:dbl[])  [unwired: 1 out]
        n2853 = call "downsample 1D array - double.vi"("Ave N"=w4336, "Array In"=w4340) -> ("Array Out"=w4339:dbl[])  [unwired: 1 out]
        n2854 = call "downsample 1D array - double.vi"("Ave N"=w4336, "Array In"=w4345) -> ("Array Out"=w4344:dbl[])  [unwired: 1 out]
        n2855 = Multiply(x=w4249, y=u64 2) -> (x*y=w4251:u64)
        n2856 = feedback #14(w4255) -> (w4313:dbl[])
        n2857 = Build Array (concatenate)(w4313, w4255) -> (w4312:dbl[])
        n2858 = feedback #15(w4247) -> (w4248:dbl[])
        n2859 = Build Array (concatenate)(w4248, w4247) -> (w4246:dbl[])
        n2860 = Select(t=w4255, s=w4253, f=w4312) -> (s? t:f=w4297:dbl[])
        n2861 = feedback-in #14(w4297) -> ()
        n2862 = Select(t=w4247, s=w4253, f=w4246) -> (s? t:f=w4271:dbl[])
        n2863 = feedback-in #15(w4271) -> ()
        n2864 = feedback #16(w4257) -> (w4406:dbl[])
        n2865 = Build Array (concatenate)(w4406, w4257) -> (w4388:dbl[])
        n2866 = Select(t=w4257, s=w4253, f=w4388) -> (s? t:f=w4392:dbl[])
        n2867 = feedback-in #16(w4392) -> ()
        n2868 = feedback #17(w4337) -> (w4394:dbl[])
        n2869 = Build Array (concatenate)(w4394, w4337) -> (w4385:dbl[])
        n2870 = feedback #18(w4344) -> (w4404:dbl[])
        n2871 = Build Array (concatenate)(w4404, w4344) -> (w4403:dbl[])
        n2872 = feedback #19(w4339) -> (w4396:dbl[])
        n2873 = Build Array (concatenate)(w4396, w4339) -> (w4397:dbl[])
        n2874 = Select(t=w4337, s=w4253, f=w4385) -> (s? t:f=w4341:dbl[])
        n2875 = feedback-in #17(w4341) -> ()
        n2876 = Select(t=w4344, s=w4253, f=w4403) -> (s? t:f=w4343:dbl[])
        n2877 = feedback-in #18(w4343) -> ()
        n2878 = Select(t=w4339, s=w4253, f=w4397) -> (s? t:f=w4342:dbl[])
        n2879 = feedback-in #19(w4342) -> ()
        n2880 = call "integrate 1D array interval - double.vi"("Ave N"=w4252, "Array In"=w4297) -> ("Array Out"=w4308:dbl[])  [unwired: 1 out]
        n2881 = call "integrate 1D array interval - double.vi"("Ave N"=w4252, "Array In"=w4271) -> ("Array Out"=w4282:dbl[])  [unwired: 1 out]
        n2882 = call "integrate 1D array interval - double.vi"("Ave N"=w4252, "Array In"=w4392) -> ("Array Out"=w4391:dbl[])  [unwired: 1 out]
        n2883 = Array Size(array=w4308) -> (size(s)=w4309:i32)
        n2884 = Array Size(array=w4282) -> (size(s)=w4283:i32)
        n2885 = Array Size(array=w4391) -> (size(s)=w4393:i32)
        n2886 = Multiply(x=w4250, y=w4251) -> (x*y=w4311:u64)
        n2887 = Multiply(x=w4250, y=w4251) -> (x*y=w4285:u64)
        n2888 = Multiply(x=w4250, y=w4251) -> (x*y=w4401:u64)
        n2889 = Subtract(x=w4311, y=w4309) -> (x-y=w4302:u64)
        n2890 = call-poly <vilib>:"Mean.vi"("X"=w4308) -> ("mean"=w4299:dbl)  [unwired: 1 out]
        n2891 = Subtract(x=w4285, y=w4283) -> (x-y=w4276:u64)
        n2892 = call-poly <vilib>:"Mean.vi"("X"=w4282) -> ("mean"=w4273:dbl)  [unwired: 1 out]
        n2893 = Subtract(x=w4401, y=w4393) -> (x-y=w4335:u64)
        n2894 = call-poly <vilib>:"Mean.vi"("X"=w4391) -> ("mean"=w4332:dbl)  [unwired: 1 out]
        n2895 = call-poly <vilib>:"Mean.vi"("X"=w4341) -> ("mean"=w4325:dbl)  [unwired: 1 out]
        n2896 = call-poly <vilib>:"Mean.vi"("X"=w4343) -> ("mean"=w4330:dbl)  [unwired: 1 out]
        n2897 = call-poly <vilib>:"Mean.vi"("X"=w4342) -> ("mean"=w4328:dbl)  [unwired: 1 out]
        n2898 = Initialize Array(1.0 ("element"), w4302) -> (w4298:dbl[])
        n2899 = Initialize Array(1.0 ("element"), w4276) -> (w4272:dbl[])
        n2900 = Initialize Array(1.0 ("element"), w4335) -> (w4326:dbl[])
        n2901 = Multiply(x=w4298, y=w4299) -> (x*y=w4300:dbl[])
        n2902 = Multiply(x=w4272, y=w4273) -> (x*y=w4274:dbl[])
        n2903 = Multiply(x=w4326, y=w4332) -> (x*y=w4333:dbl[])
        n2904 = Multiply(x=w4326, y=w4328) -> (x*y=w4329:dbl[])
        n2905 = Multiply(x=w4326, y=w4330) -> (x*y=w4331:dbl[])
        n2906 = Multiply(x=w4326, y=w4325) -> (x*y=w4327:dbl[])
        n2907 = Build Array (concatenate)(w4308, w4300) -> (w4310:dbl[])
        n2908 = Build Array (concatenate)(w4282, w4274) -> (w4284:dbl[])
        n2909 = Build Array (concatenate)(w4391, w4333) -> (w4400:dbl[])
        n2910 = Build Array (concatenate)(w4341, w4327) -> (w4395:dbl[])
        n2911 = Build Array (concatenate)(w4343, w4331) -> (w4399:dbl[])
        n2912 = Build Array (concatenate)(w4342, w4329) -> (w4398:dbl[])
        n2913 = Reshape Array(w4310, w4250, w4251) -> (w4306:dbl[][])
        n2914 = Reshape Array(w4284, w4250, w4251) -> (w4280:dbl[][])
        n2915 = Reshape Array(w4400, w4250, w4251) -> (w4378:dbl[][])
        n2916 = Reshape Array(w4395, w4250, w4251) -> (w4361:dbl[][])
        n2917 = Reshape Array(w4399, w4250, w4251) -> (w4353:dbl[][])
        n2918 = Reshape Array(w4398, w4250, w4251) -> (w4368:dbl[][])
        n2919 = Array Subset(array=w4306, index (col)=0 ("index"), length (col)=w4249) -> (w4305:dbl[][])  [unwired: 2 in]
        n2920 = Array Subset(array=w4306, index (col)=w4249) -> (w4303:dbl[][])  [unwired: 3 in]
        n2921 = Array Subset(array=w4280, index (col)=0 ("index"), length (col)=w4249) -> (w4279:dbl[][])  [unwired: 2 in]
        n2922 = Array Subset(array=w4280, index (col)=w4249) -> (w4277:dbl[][])  [unwired: 3 in]
        n2923 = Array Subset(array=w4368, index (col)=0 ("index"), length (col)=w4249) -> (w4373:dbl[][])  [unwired: 2 in]
        n2924 = Array Subset(array=w4368, index (col)=w4249) -> (w4371:dbl[][])  [unwired: 3 in]
        n2925 = Array Subset(array=w4378, index (col)=0 ("index"), length (col)=w4249) -> (w4377:dbl[][])  [unwired: 2 in]
        n2926 = Array Subset(array=w4378, index (col)=w4249) -> (w4375:dbl[][])  [unwired: 3 in]
        n2927 = Array Subset(array=w4353, index (col)=0 ("index"), length (col)=w4249) -> (w4359:dbl[][])  [unwired: 2 in]
        n2928 = Array Subset(array=w4353, index (col)=w4249) -> (w4357:dbl[][])  [unwired: 3 in]
        n2929 = Array Subset(array=w4361, index (col)=0 ("index"), length (col)=w4249) -> (w4366:dbl[][])  [unwired: 2 in]
        n2930 = Array Subset(array=w4361, index (col)=w4249) -> (w4364:dbl[][])  [unwired: 3 in]
        n2931 = for {
          tunnel: w4305 -> [w4410] mode=indexing
          tunnel: [w4409] -> w4304 mode=indexing
          workers-P: _ -> [_]
          n2932 = Reverse 1D Array(array=w4410) -> (reversed array=w4409:dbl[])
        }
        n2933 = for {
          tunnel: w4279 -> [w4408] mode=indexing
          tunnel: [w4407] -> w4278 mode=indexing
          workers-P: _ -> [_]
          n2934 = Reverse 1D Array(array=w4408) -> (reversed array=w4407:dbl[])
        }
        n2935 = for {
          tunnel: w4373 -> [w4416] mode=indexing
          tunnel: [w4415] -> w4372 mode=indexing
          workers-P: _ -> [_]
          n2936 = Reverse 1D Array(array=w4416) -> (reversed array=w4415:dbl[])
        }
        n2937 = for {
          tunnel: w4377 -> [w4418] mode=indexing
          tunnel: [w4417] -> w4376 mode=indexing
          workers-P: _ -> [_]
          n2938 = Reverse 1D Array(array=w4418) -> (reversed array=w4417:dbl[])
        }
        n2939 = for {
          tunnel: w4359 -> [w4412] mode=indexing
          tunnel: [w4411] -> w4358 mode=indexing
          workers-P: _ -> [_]
          n2940 = Reverse 1D Array(array=w4412) -> (reversed array=w4411:dbl[])
        }
        n2941 = for {
          tunnel: w4366 -> [w4414] mode=indexing
          tunnel: [w4413] -> w4365 mode=indexing
          workers-P: _ -> [_]
          n2942 = Reverse 1D Array(array=w4414) -> (reversed array=w4413:dbl[])
        }
        n2943 = Index Array(array=w4378, index (row)=0) -> (element=→"Waveform Graph":dbl[])  [unwired: 1 in]
        n2944 = Add(x=w4304, y=w4303) -> (x+y=w4290:dbl[][])
        n2945 = Add(x=w4278, y=w4277) -> (x+y=w4264:dbl[][])
        n2946 = Add(x=w4372, y=w4371) -> (x+y=w4370:dbl[][])
        n2947 = Add(x=w4376, y=w4375) -> (x+y=w4350:dbl[][])
        n2948 = Add(x=w4358, y=w4357) -> (x+y=w4356:dbl[][])
        n2949 = Add(x=w4365, y=w4364) -> (x+y=w4363:dbl[][])
        n2950 = Divide(x=w4356, y=2) -> (x/y=w4354:dbl[][])
        n2951 = Divide(x=w4370, y=2) -> (x/y=w4315:dbl[][])
        n2952 = To Single Precision Float(number=w4350) -> (single precision float=w4349:sgl[][])
        n2953 = To Single Precision Float(number=w4290) -> (single precision float=w4294:sgl[][])
        n2954 = To Single Precision Float(number=w4264) -> (single precision float=w4268:sgl[][])
        n2955 = Divide(x=w4363, y=2) -> (x/y=w4317:dbl[][])
        n2956 = Transpose 2D Array(2D array=w4354) -> (transposed array=→"Data map":dbl[][])
        n2957 = To Single Precision Float(number=w4315) -> (single precision float=w4321:sgl[][])
        n2958 = To Single Precision Float(number=w4317) -> (single precision float=w4318:sgl[][])
        n2959 = call "IMAQ ArrayToImage"("Image Pixels (Float)"=w4349, "Image"=w4287) -> ("Image Out"=w4352:T2)  [unwired: 8 in, 1 out]
        n2960 = call "IMAQ ArrayToImage"("Image Pixels (Float)"=w4294, "Image"=w4286) -> ("Image Out"=w4296:T2)  [unwired: 8 in, 1 out]
        n2961 = call "IMAQ ArrayToImage"("Image Pixels (Float)"=w4268, "Image"=w4260) -> ("Image Out"=w4270:T2)  [unwired: 8 in, 1 out]
        n2962 = call "IMAQ ArrayToImage"("Image Pixels (Float)"=w4321, "Image"=w4261) -> ("Image Out"=w4323:T2)  [unwired: 8 in, 1 out]
        n2963 = call "IMAQ Symmetry"("Type of Symmetry"=w4351, "Image Src"=w4352) -> ("Image Dst Out"=w4347:T2)  [unwired: 3 in, 1 out]
        n2964 = call "IMAQ ArrayToImage"("Image Pixels (Float)"=w4318, "Image"=w4262) -> ("Image Out"=w4320:T2)  [unwired: 8 in, 1 out]
        n2965 = call "IMAQ Symmetry"("Type of Symmetry"=w4295, "Image Src"=w4296) -> ("Image Dst Out"=w4292:T2)  [unwired: 3 in, 1 out]
        n2966 = call "IMAQ Symmetry"("Type of Symmetry"=w4269, "Image Src"=w4270) -> ("Image Dst Out"=w4266:T2)  [unwired: 3 in, 1 out]
        n2967 = call "IMAQ Symmetry"("Type of Symmetry"=w4322, "Image Src"=w4323) -> ("Image Dst Out"=→"Detection Laser X":T2)  [unwired: 3 in, 1 out]
        n2968 = call "IMAQ Symmetry"("Type of Symmetry"=w4319, "Image Src"=w4320) -> ("Image Dst Out"=→"Detection Laser Y":T2)  [unwired: 3 in, 1 out]
        n2969 = call "IMAQ Set Simple Calibration"("Calibration Axis Info"=T39 {"Origin Pixel"={"X"=0.0, "Y"=0.0}, "Angle Relative to Horizontal (deg)"=0.0, "Axis Reference"=0}, "Grid Descriptor"=T40 {"X Step"=0.3, "Y Step"=0.3, "Unit"=enum."Undefined"}, "Image"=w4347) -> ("Calibrated Image"=→"APD 1":T2)  [unwired: 7 in, 1 out]
        n2970 = call "IMAQ Set Simple Calibration"("Calibration Axis Info"=T39 {"Origin Pixel"={"X"=0.0, "Y"=0.0}, "Angle Relative to Horizontal (deg)"=0.0, "Axis Reference"=0}, "Grid Descriptor"=T40 {"X Step"=0.3, "Y Step"=0.3, "Unit"=enum."Undefined"}, "Image"=w4292) -> ("Calibrated Image"=→"APD 2":T2)  [unwired: 7 in, 1 out]
        n2971 = call "IMAQ Set Simple Calibration"("Calibration Axis Info"=T39 {"Origin Pixel"={"X"=0.0, "Y"=0.0}, "Angle Relative to Horizontal (deg)"=0.0, "Axis Reference"=0}, "Grid Descriptor"=T40 {"X Step"=0.3, "Y Step"=0.3, "Unit"=enum."Undefined"}, "Image"=w4266) -> ("Calibrated Image"=→"APD 3":T2)  [unwired: 7 in, 1 out]
      }
    }
    n2972 = case "For computing FFTs for display" shown="True" "Compute FFT" {
      tunnel: w3748 -> [_ w4890]
      frame False {
      }
      frame True {
        n2973 = Build Array("FFT 1 Choice 1", "FFT 1 Choice 2", "FFT 2 Choice 1", "FFT 2 Choice 2") -> (w4883:u16[])
        n2974 = Array Size(array=w4890) -> (size(s)=w4889:i32)
        n2975 = feedback-in #20(w4883) -> ()
        n2976 = feedback #20(u16[] [100, 100, 100, 100]) -> (w4884:u16[])
        n2977 = feedback-in #21("# Spectra to Ave.") -> ()
        n2978 = feedback #21("# Spectra to Ave.") -> (w4881:dbl)
        n2979 = Not Equal?(x="# Spectra to Ave.", y=w4881) -> (x != y?=w4880:bool)
        n2980 = Not Equal?(x=w4883, y=w4884) -> (x != y?=w4882:bool)
        n2981 = feedback #22(1.0) -> (w4867:dbl)
        n2982 = Compound Arithmetic op=OR("Reset FFT", w4882, w4880) -> (w4865:bool)
        n2983 = Select(t=1.0, s=w4865, f=w4867) -> (s? t:f=w4869:dbl)
        n2984 = Greater?(x=w4869, y="# Spectra to Ave.") -> (0:w4888:bool)
        n2985 = Increment(x=w4869) -> (x+1=w4868:dbl)
        n2986 = feedback-in #22(w4868) -> ()
        n2987 = local read "DMA Update Period (s)"() -> (w4863:dbl)
        n2988 = Multiply(x="# Spectra to Ave.", y=w4863) -> (x*y=→"Ave. Time (s)":dbl)
        n2989 = Build Array(cluster{"f0":dbl, "df":dbl, "magnitude":dbl[]} {"f0"=0.0, "df"=0.0, "magnitude"=[]} ("PSD")) -> (w4872:cluster{"f0":dbl, "df":dbl, "magnitude":dbl[]}[])
        n2990 = Build Array(w4872, w4872, w4872, w4872) -> (w4874:T49)
        n2991 = feedback #23(w4874) -> (w4879:T49)
        n2992 = for {
          N: 4 -> [_]
          tunnel: w4883 -> [w4912] mode=indexing
          tunnel: w4890 -> [w4913]
          tunnel: w4889 -> [w4915]
          tunnel: w4865 -> [w4908]
          tunnel: w4888 -> [w4907]
          tunnel: "# Spectra to Ave." -> [w4906]
          tunnel: [w4905] -> w4878 mode=indexing
          tunnel: w4879 -> [w4910] mode=indexing
          tunnel: [w4909] -> w4866 mode=indexing
          tunnel: w4869 -> [w4904]
          n2993 = Less?(x=w4912, y=w4915) -> (x < y?=w4914:bool)
          n2994 = Index Array(array=w4913, index=w4912) -> (element=w4911:waveform(dbl))
          n2995 = case shown="True" w4914 {
            tunnel: w4911 -> [_ w4932]
            tunnel: w4910 -> [w4917 w4930]
            tunnel: [w4917 w4918] -> w4909
            tunnel: w4908 -> [_ w4929]
            tunnel: w4907 -> [_ w4922]
            tunnel: w4906 -> [_ w4921]
            tunnel: [cluster{"f0":dbl, "df":dbl, "magnitude":dbl[]} {"f0"=0.0, "df"=0.0, "magnitude"=[]} ("PSD") w4923] -> w4905
            tunnel: w4904 -> [_ w4920]
            frame False {
            }
            frame True {
              n2996 = call <vilib>:"Std Deviation and Variance.vi"("X"=w4932) -> ("mean"=w4933:dbl)  [unwired: 1 in, 2 out]
              n2997 = Subtract(x=w4932, y=w4933) -> (x-y=w4931:waveform(dbl))
              n2998 = xnode "Spectral Measurements"("Signals"=w4931) -> ("PSD"=w4925:cluster{"f0":dbl, "df":dbl, "magnitude":dbl[]})  [unwired: 1 in, 1 out]
              n2999 = case shown="False" w4929 {
                tunnel: w4930 -> [w4942 _]
                tunnel: [w4938 w4947] -> w4918
                tunnel: w4925 -> [w4941 w4948]
                tunnel: w4922 -> [w4940 _]
                frame False {
                  n3000 = Build Array (concatenate)(w4942, w4941) -> (w4939:cluster{"f0":dbl, "df":dbl, "magnitude":dbl[]}[])
                  n3001 = case shown="True" w4940 {
                    tunnel: w4939 -> [w4943 w4946]
                    tunnel: [w4943 w4944] -> w4938
                    frame False {
                    }
                    frame True {
                      n3002 = Delete From Array(array=w4946, index=0) -> (array with subset deleted=w4944:cluster{"f0":dbl, "df":dbl, "magnitude":dbl[]}[])  [unwired: 1 in, 1 out]
                    }
                  }
                }
                frame True {
                  n3003 = Build Array(w4948) -> (w4947:cluster{"f0":dbl, "df":dbl, "magnitude":dbl[]}[])
                }
              }
              n3004 = for {
                tunnel: w4918 -> [w4937] mode=indexing
                tunnel: [w4936] -> w4928 mode=indexing
                workers-P: _ -> [_]
                n3005 = Unbundle By Name(w4937) -> ("magnitude"=w4936:dbl[])
              }
              n3006 = Transpose 2D Array(2D array=w4928) -> (transposed array=w4927:dbl[][])
              n3007 = for {
                tunnel: w4927 -> [w4935] mode=indexing
                tunnel: [w4934] -> w4926 mode=indexing
                workers-P: _ -> [_]
                n3008 = Add Array Elements(numeric array=w4935) -> (sum=w4934:dbl)
              }
              n3009 = Select(t=w4921, s=w4922, f=w4920) -> (s? t:f=w4919:dbl)
              n3010 = Divide(x=w4926, y=w4919) -> (x/y=w4924:dbl[])
              n3011 = Bundle By Name(cluster=w4925, "magnitude"=w4924) -> (w4923:cluster{"f0":dbl, "df":dbl, "magnitude":dbl[]})
            }
          }
        }
        n3012 = case shown="True" w4865 {
          tunnel: w4866 -> [w4897 w4903]
          tunnel: [w4897 w4898] -> w4864
          frame False {
          }
          frame True {
            n3013 = Array Subset(array=w4903, index (row)=0 ("index"), length (row)=4 ("length"), index (col)=0 ("index"), length (col)=1 ("length")) -> (w4898:T49)
          }
        }
        n3014 = feedback-in #23(w4864) -> ()
        n3015 = Split 1D Array(array=w4878, index=2) -> (first subarray=→"FFT 1":cluster{"f0":dbl, "df":dbl, "magnitude":dbl[]}[], second subarray=→"FFT 2":cluster{"f0":dbl, "df":dbl, "magnitude":dbl[]}[])
      }
    }
    n3016 = Divide(x="T1 offset_x (mV)", y=1000.0) -> (x/y=w3799:dbl)
    n3017 = feedback-in #24("Calibration") -> ()
    n3018 = feedback #24(u16 1 ("Calibration")) -> (w3817:u16)
    n3019 = Divide(x="T2 offset_x (mV)", y=1000.0) -> (x/y=w3798:dbl)
    n3020 = case shown="2" "Calibration" {
      tunnel: "T1 alpha_x (nm/V)" -> [_ w4208 w4232]
      tunnel: "T1 kappa_x (pN/nm)" -> [_ _ w4222]
      tunnel: "T2 alpha_x (nm/V)" -> [_ w4207 w4230]
      tunnel: "T2 kappa_x (pN/nm)" -> [_ _ w4223]
      tunnel: w3553 -> [w4187 w4205 w4228]
      tunnel: w3552 -> [w4186 w4203 w4226]
      tunnel: [w4187 w4202 w4225] -> w3826
      tunnel: [w4186 w4201 w4224] -> w3825
      tunnel: [w4181 w4191 w4214] -> w3814
      tunnel: [w4178 w4190 w4213] -> w3813
      tunnel: ["Position (V)" ("Label.Text") "Position (nm)" ("Label.Text") "Force (pN)" ("Label.Text")] -> w3815
      tunnel: w3798 -> [_ w4195 w4217]
      tunnel: w3799 -> [_ w4198 w4219]
      tunnel: ["Mean (V)" ("Label.Text") "Mean (nm)" ("Label.Text") "Mean (pN)" ("Label.Text")] -> w3810
      tunnel: ["Difference (V)" ("Label.Text") "Difference (nm)" ("Label.Text") "Difference (pN)" ("Label.Text")] -> w3754
      tunnel: w3551 -> [w4182 w4189 w4211]
      tunnel: w3550 -> [w4179 w4188 w4210]
      frame 0, Default {
        w4180 = " (V)" ("Label.Text")
        n3021 = Concatenate Strings(w4182, w4180) -> (w4181:string)
        n3022 = Concatenate Strings(w4179, w4180) -> (w4178:string)
      }
      frame 1 {
        w4192 = " (nm)" ("Label.Text")
        n3023 = Unbundle By Name(w4205) -> ("Y"=w4209:dbl[])
        n3024 = Unbundle By Name(w4203) -> ("Y"=w4196:dbl[])
        n3025 = Subtract(x=w4209, y=w4198) -> (x-y=w4199:dbl[])
        n3026 = Subtract(x=w4196, y=w4195) -> (x-y=w4197:dbl[])
        n3027 = Multiply(x=w4197, y=w4207) -> (x*y=w4204:dbl[])
        n3028 = Multiply(x=w4208, y=w4199) -> (x*y=w4206:dbl[])
        n3029 = Bundle By Name(cluster=w4203, "Y"=w4204) -> (w4201:waveform(dbl))
        n3030 = Bundle By Name(cluster=w4205, "Y"=w4206) -> (w4202:waveform(dbl))
        n3031 = Concatenate Strings(w4189, w4192) -> (w4191:string)
        n3032 = Concatenate Strings(w4188, w4192) -> (w4190:string)
      }
      frame 2 {
        w4212 = " (pN)" ("Label.Text")
        n3033 = Unbundle By Name(w4228) -> ("Y"=w4233:dbl[])
        n3034 = Unbundle By Name(w4226) -> ("Y"=w4231:dbl[])
        n3035 = Subtract(x=w4231, y=w4217) -> (x-y=w4218:dbl[])
        n3036 = Subtract(x=w4233, y=w4219) -> (x-y=w4220:dbl[])
        n3037 = Compound Arithmetic op=MULTIPLY(w4218, w4230, w4223) -> (w4227:dbl[])
        n3038 = Compound Arithmetic op=MULTIPLY(w4222, w4232, w4220) -> (w4229:dbl[])
        n3039 = Bundle By Name(cluster=w4226, "Y"=w4227) -> (w4224:waveform(dbl))
        n3040 = Bundle By Name(cluster=w4228, "Y"=w4229) -> (w4225:waveform(dbl))
        n3041 = Concatenate Strings(w4210, w4212) -> (w4213:string)
        n3042 = Concatenate Strings(w4211, w4212) -> (w4214:string)
      }
    }
    n3043 = case shown="True" "Read Lateness and Rel Phase" {
      tunnel: w3621 -> [w4139 w4172]
      tunnel: w3620 -> [w4140 w4171]
      tunnel: [w4139 w4144] -> w3794
      tunnel: [w4140 w4143] -> w3793
      frame False {
      }
      frame True {
        n3044 = xnode "Read/Write Control"("FPGA VI Reference In"=w4172, "error in"=w4171) -> ("FPGA VI Reference Out"=w4146:T20, "error out"=w4145:errorcluster, "GI Relative phase"=→"GI relative phase":i16, "Relative phase"=→"Relative phase (AI1)":i16, "AI Late Counter"=→"Late Counter (AI1)":u8, "GI Late Counter"=→"GI Late Counter":u8, "MCL Late Counter"=→"MCL Late Counter":u8, "MCL Relative Phase"=→"Relative Phase (MCL)":i16, "APD Acq Relative Phase"=→"APD Acq Relative Phase":i16, "APD 1 Gate Relative Phase"=→"APD 1 Gate Relative Phase":i16, "APD 2 Gate Relative Phase"=→"APD 2 Gate Relative Phase":i16, "APD Acq Late Counter"=→"APD Acq Late Counter":u8, "APD 1 Gate Late Counter"=→"APD 1 Gate Late Counter":u8, "APD 2 Gate Late Counter"=→"APD 2 Gate Late Counter":u8, "Green FB Relative Phase"=→"Relative phase (Green FB)":i16, "GI Relative phase 2"=→"GI relative phase 2":i16, "GI Late Counter 2"=→"GI Late Counter 2":u8, "Trap Pos FIFO Timeout"=→"Trap Pos FIFO Timeout":u16, "Trap AI FIFO Timeout"=→"Trap AI FIFO Timeout":u16, "RI Late Counter"=→"RI Late Counter":u8, "RI Relative phase"=→"RI relative phase":i16, "Green Late Counter"=→"Green AI Late Counter":u8, "BI Late Counter (AO)"=→"Late Counter (BI AO)":u8, "Blue Late Counter (D)"=→"Late Counter (BI DO)":u8, "BI Relative phase (AO)"=→"Relative phase (BI AO)":i16, "BI Relative phase (D)"=→"Relative phase (BI DO)":i16)